vi "CRYO_MASTER_FULL_RUN3.vi"() -> ()   [LabVIEW 2017] (continued)
  T14 = enum16{"N.C.", "T3He1-1", "T3He1-2", "T3He1-3", "T3He1-4", "T3He2-1", "T3He2-2", "T3He3", "T3He4", "T3He5", "T3He6-1", "T3He6-2", "T3He7-1", "T3He7-2", "T3He8", "T3He9", "T3He10", "T4He1", "T4He2-1", "T4He2-2", "T4He3-1", "T4He3-2", "T4He3-3", "T4He3-4", "T4He4", "T4He5", "T4He6", "T4He7", "T4He8", "T4He9", "T4He10", "T1K1", "T1K2", "T1K3-1", "T1K3-2", "T1K4", "T1K5", "T1K6", "TIP1", "TIP2", "TIP3", "TIP4", "TIP5", "TIP6", "TIP7", "TTH1", "TTH2", "TTH3", "TTH4"}
  T15 = cluster{"Source":enum16{"USB6210", "USB6218AI", "USB6218AO", "LSI218", "LSI336", "DMMs"}, "SourceLabel":string}
  T16 = cluster{"Source":enum16{"USB6210", "USB6218AI", "USB6218AO", "LSI218", "LSI336", "DMMs"}, "SourceLabel":string, "FileFormat":string}[]
  T17 = cluster{"LSIName":string, "Active?":bool, "LastData":dbl[], "Labels":string[]}[]
  T18 = enum16{"N.C.", "T3He1-1", "T3He1-2", "T3He1-3", "T3He1-4", "T3He2-1", "T3He2-2", "T3He3", "T3He4", "T3He5", "T3He6-1", "T3He6-2", "T3He7-1", "T3He7-2", "T3He8", "T3He9", "T3He10", "T4He1", "T4He2-1", "T4He2-2", "T4He3-1", "T4He3-2", "T4He3-3", "T4He3-4", "T4He4", "T4He5", "T4He6", "T4He7", "T4He8", "T4He9", "T4He10", "T1K1", "T1K2", "T1K3-1", "T1K3-2", "T1K4", "T1K5", "T1K6", "TIP1", "TIP2", "TIP3", "TIP4", "TIP5", "TIP6", "TIP7", "TTH1", "TTH2", "TTH3", "TTH4"}[]
  T19 = cluster{"TimeArray (USB6218)":timestamp[], "DataArrayConv (USB6218)":dbl[]}
  T20 = cluster{"appended array":timestamp[], "ActualCurrentArray":dbl[]}
  T21 = cluster{"appended array":timestamp[], "SetCurrentArray":dbl[]}
  T22 = cluster{"appended array":timestamp[], "SetCurrentArray":dbl[]}[]
  T23 = typedef "imagedata.ctl" = cluster{"image type":i32, "image depth":i32, "image":u8[], "mask":u8[], "colors":u32[], "Rectangle":cluster{"left":i16, "top":i16, "right":i16, "bottom":i16}}
  T24 = enum16{"open", "replace", "create", "open or create", "replace or create", "replace or create with confirmation"}
  T25 = cluster{"TimeArray":timestamp[], "DataArrayConv":dbl[]}[]
  T26 = cluster{"IndexArray":i64[], "TimeArray":timestamp[], "DataArrayRaw":dbl[][], "DataArrayConv":dbl[][], "LDArray":dbl[]}
  T27 = cluster{"InstName":string, "Active?":bool, "Status":enum16{"Intialized", "Ready", "Measuring", "Terminated"}, "Labels":string[], "LabelLD":string, "FileFormat":string[], "FileFormatLD":string, "ReadLeakDet?":bool}
  T28 = cluster{"AOUT Labels[0]":string, "AOUT Labels[1]":string, "AOUT Labels[2]":string, "AOUT Labels[3]":string, "AOUT Labels[4]":string, "AOUT Labels[5]":string, "AOUT Labels[6]":string, "AOUT Labels[7]":string, "AOUT Labels[8]":string}
  T29 = cluster{"LastTimeArray":timestamp[], "LastDataArray":dbl[]}
  T30 = cluster{"LastTimeArray":timestamp[], "LastDataArray":dbl[]}[]
  T31 = cluster{"TimeArray":timestamp[], "DataArrayConv":dbl[]}
  T32 = cluster{"TimeArray":timestamp[], "DataArrayConv (USB6218)":dbl[]}
  T33 = cluster{"TimeArray":timestamp[], "M.A. Array":dbl[]}
  T34 = cluster{"TimeArray":timestamp[], "M.A. Array":dbl[]}[]
  T35 = cluster{"TimeArray":timestamp[], "DataArray":dbl[]}
  T36 = enum16{"USB6210", "USB6218AI", "USB6218AO", "LSI218", "LSI336", "DMMs"}
diagram:
  w17 = TRUE ("create if not found? (T)")
  w21 = errorcluster {"status"=FALSE, "code"=0, "source"=""} ("error in (no error)")
  w6 = errorcluster {"status"=FALSE, "code"=0, "source"=""} ("error in (no error)")
  n1 = while {
    shift-right: [w44] -> _
    shift-left: dbl[] [] -> [w50]
    shift-right: [w47] -> _
    shift-left: timestamp[] [] -> [w49]
    i -> [w48]
    stop <- w51 stop-if-true
    n2 = Wait (ms)(milliseconds to wait=u32 225) -> ()  [unwired: 1 out]
    n3 = event shown="[6] \"OUTPUT (PWR)\", \"OUTPUT (PMC)\": Value Change" {
      selector: _ -> [_ _ _ _ _ _ _]
      dyn-events: _ -> [_ _ _ _ _ _ _]
      timeout: _ -> [_ _ _ _ _ _ _]
      tunnel: [_ TRUE _ _ _ _ _] -> w51
      tunnel: w48 -> [_ _ _ _ w132 _ _]
      tunnel: [_ _ _ _ w131 w215 _] -> w44
      tunnel: w50 -> [_ _ _ _ w128 w215 _]
      tunnel: [w53 w63 _ _ w130 w214 w218] -> w47
      tunnel: w49 -> [w53 w63 _ _ w129 w214 w218]
      tunnel: w48 -> [_ _ w69 w93 _ _ w219]
      tunnel: [_ _ _ _ w119 _ _] -> w43
      event Timeout {
        n4 = event-data() -> ()  [unwired: 1 in, 3 out]
      }
      event "Stop Button": Value Change {
        w54 = FALSE
        n5 = event-data() -> ()  [unwired: 1 in, 3 out]
        n6 = local read "error out (USB6210/6218 DOUT)"() -> (w62:errorcluster)
        n7 = local read "error out (USB6210/6218 AOUT)"() -> (w59:errorcluster)
        n8 = local read "DOUT task out"() -> (w58:refnum<k21>)
        n9 = local read "AO task out"() -> (w65:refnum<k21>)
        n10 = property on="OUTPUT\n(PWR)" class="Bool (strict)"("Value"=w54) -> ()  [unwired: 2 in, 2 out]
        n11 = property on="V2 (N.C.)" class="Bool (strict)"("Val(Sgnl)"=w54) -> ()  [unwired: 2 in, 2 out]
        n12 = property on="OUTPUT\n(PMC)" class="Bool (strict)"("Value"=w54) -> ()  [unwired: 2 in, 2 out]
        n13 = Build Array(w54, w54, w54, w54) -> (w61:bool[])
        n14 = Not(x=w54) -> (.not. x?=w55:bool)
        n15 = call <vilib>:"DAQmx Clear Task.vi"("task in"=w65, "error in"=w59) -> ("error out"=w64:errorcluster)  [unwired: 13 in]
        n16 = property on="V1 (N.O.)" class="Bool (strict)"("Val(Sgnl)"=w55) -> ()  [unwired: 2 in, 2 out]
        n17 = call <vilib>:"DAQmx Write (Digital 1D Bool NChan 1Samp 1Line).vi"("task/channels in"=w58, "data"=w61, "timeout"=10.0, "error in"=w62) -> ("task out"=w57:refnum<k21>, "error out"=w56:errorcluster)  [unwired: 9 in, 1 out]
        n18 = call <vilib>:"DAQmx Clear Task.vi"("task in"=w57, "error in"=w56) -> ("error out"=w66:errorcluster)  [unwired: 13 in]
        n19 = local write "error out (USB6210/6218 AOUT)"(w64) -> ()
        n20 = local write "error out (USB6210/6218 DOUT)"(w66) -> ()
      }
      event "V1 (N.O.)": Value Change {
        n21 = event-data() -> ()  [unwired: 1 in, 3 out]
        n22 = local read "Cycle #"() -> (w72:u32)
        n23 = Greater?(x=w72, y=u32 0) -> (0:w70:bool)
        n24 = case shown="True" w70 {
          tunnel: "V1 (N.O.)" -> [_ w86]
          tunnel: w69 -> [_ w81]
          frame False {
          }
          frame True {
            n25 = Not(x=w86) -> (.not. x?=w88:bool)
            n26 = property on="OUTPUT\n(PMC)" class="Bool (strict)"() -> ("Value"=w73:bool)  [unwired: 2 in, 2 out]
            n27 = local read "error out (USB6210/6218 DOUT)"() -> (w87:errorcluster)
            n28 = property on="OUTPUT\n(PWR)" class="Bool (strict)"() -> ("Value"=w84:bool)  [unwired: 2 in, 2 out]
            n29 = property on="V2 (N.C.)" class="Bool (strict)"() -> ("Value"=w85:bool)  [unwired: 2 in, 2 out]
            n30 = local read "DOUT task out"() -> (w91:refnum<k21>)
            n31 = Build Array(w88, w85, w84, w73) -> (w77:bool[])
            n32 = local read "File Refn USB DO"() -> (w82:refnum<file>)
            n33 = Boolean To (0,1)(Boolean=w77) -> (0, 1=w76:i16[])
            n34 = Initialize Array("%d" ("element"), 3 ("dimension size")) -> (w80:string[])
            n35 = call <vilib>:"DAQmx Write (Digital 1D Bool NChan 1Samp 1Line).vi"("task/channels in"=w91, "data"=w77, "timeout"=10.0, "error in"=w87) -> ("task out"=w89:refnum<k21>, "error out"=w75:errorcluster)  [unwired: 9 in, 1 out]
            n36 = local write "DOUT task out"(w89) -> ()
            n37 = Get Date/Time In Seconds() -> (seconds since 1Jan1904=w83:timestamp)
            n38 = call "FileWrite.vi"("DataArray"=w76, "Time Stamp"=w83, "Error In"=w75, "FileFormat"=w80, "Index"=w81, "refnum in"=w82) -> ("Error Out"=w74:errorcluster)  [unwired: 4 in, 1 out]
            n39 = local write "error out (USB6210/6218 DOUT)"(w74) -> ()
          }
        }
        "V1" <- "V1 (N.O.)"
      }
      event "V2 (N.C.)": Value Change {
        n40 = event-data() -> ()  [unwired: 1 in, 3 out]
        n41 = local read "Cycle #"() -> (w96:u32)
        n42 = Greater?(x=w96, y=u32 0) -> (0:w94:bool)
        n43 = case shown="True" w94 {
          tunnel: "V2 (N.C.)" -> [_ w111]
          tunnel: w93 -> [_ w103]
          frame False {
          }
          frame True {
            n44 = property on="OUTPUT\n(PMC)" class="Bool (strict)"() -> ("Value"=w97:bool)  [unwired: 2 in, 2 out]
            n45 = property on="V1 (N.O.)" class="Bool (strict)"() -> ("Value"=w110:bool)  [unwired: 2 in, 2 out]
            n46 = Not(x=w110) -> (.not. x?=w109:bool)
            n47 = local read "error out (USB6210/6218 DOUT)"() -> (w114:errorcluster)
            n48 = property on="OUTPUT\n(PWR)" class="Bool (strict)"() -> ("Value"=w108:bool)  [unwired: 2 in, 2 out]
            n49 = local read "DOUT task out"() -> (w115:refnum<k21>)
            n50 = Build Array(w109, w111, w108, w97) -> (w106:bool[])
            n51 = local read "File Refn USB DO"() -> (w107:refnum<file>)
            n52 = Boolean To (0,1)(Boolean=w106) -> (0, 1=w105:i16[])
            n53 = Initialize Array("%d" ("element"), 3 ("dimension size")) -> (w100:string[])
            n54 = call <vilib>:"DAQmx Write (Digital 1D Bool NChan 1Samp 1Line).vi"("task/channels in"=w115, "data"=w106, "timeout"=10.0, "error in"=w114) -> ("task out"=w112:refnum<k21>, "error out"=w99:errorcluster)  [unwired: 9 in, 1 out]
            n55 = local write "DOUT task out"(w112) -> ()
            n56 = Get Date/Time In Seconds() -> (seconds since 1Jan1904=w104:timestamp)
            n57 = call "FileWrite.vi"("DataArray"=w105, "Time Stamp"=w104, "Error In"=w99, "FileFormat"=w100, "Index"=w103, "refnum in"=w107) -> ("Error Out"=w98:errorcluster)  [unwired: 4 in, 1 out]
            n58 = local write "error out (USB6210/6218 DOUT)"(w98) -> ()
          }
        }
        "V2" <- "V2 (N.C.)"
      }
      event "Set Current (mA)\n (PMC)", "Set Current (mA)\n (PWR)", "update current": Value Change {
        n59 = event-data() -> ()  [unwired: 1 in, 3 out]
        n60 = case shown="True" "CONTROL KIKUSUI?" {
          tunnel: w132 -> [_ w183]
          tunnel: [w142 w176] -> w131
          tunnel: [w145 w175] -> w130
          tunnel: w129 -> [w147 w178]
          tunnel: w128 -> [w143 w177]
          tunnel: "Set Current (mA)\n (PWR)" -> [_ w155]
          tunnel: "Set Current (mA)\n (PMC)" -> [_ w159]
          frame False {
            w144 = 0.0 ("element")
            n61 = Get Date/Time In Seconds() -> (seconds since 1Jan1904=w146:timestamp)
            n62 = local read "AO task out"() -> (w152:refnum<k21>)
            n63 = Build Array (concatenate)(w147, w146) -> (w145:timestamp[])
            n64 = Build Array (concatenate)(w143, w144) -> (w142:dbl[])
            n65 = Build Array(w144, w144) -> (w150:dbl[])
            n66 = call <vilib>:"DAQmx Write (Analog 1D DBL NChan 1Samp).vi"("task/channels in"=w152, "data"=w150, "timeout"=100.0, "error in"=errorcluster {"status"=FALSE, "code"=0, "source"=""}) -> ("task out"=w153:refnum<k21>, "error out"=w148:errorcluster)  [unwired: 9 in, 1 out]
            n67 = local write "AO task out"(w153) -> ()
            n68 = local write "error out (KIKUSI CTRL)"(w148) -> ()
          }
          frame True {
            w170 = 2 ("index")
            n69 = xnode "Formula"("X1"=w155) -> ("Result"=w172:dbl)  [unwired: 1 in, 1 out]
            n70 = xnode "Formula"("X1"=w159) -> ("Result"=w166:dbl)  [unwired: 1 in, 1 out]
            n71 = Build Array (concatenate)(w177, w155) -> (w176:dbl[])
            n72 = In Range and Coerce(upper limit=10.0, x=w172, lower limit=0.0 ("y")) -> (coerced(x)=w164:dbl, In Range?=w165:bool)
            n73 = In Range and Coerce(upper limit=10.0, x=w166, lower limit=0.0 ("y")) -> (coerced(x)=w161:dbl, In Range?=w162:bool)
            n74 = case shown="False" w165 {
              tunnel: w164 -> [_ w195]
              tunnel: [0.0 ("upper limit") w195] -> w163
              frame False {
              }
              frame True {
              }
            }
            n75 = case shown="True" w162 {
              tunnel: w161 -> [_ w193]
              tunnel: [0.0 ("upper limit") w193] -> w160
              frame False {
              }
              frame True {
              }
            }
            n76 = Multiply(x=w155, y=0.001) -> (x*y=w154:dbl)
            n77 = Multiply(x=w159, y=0.001) -> (x*y=w158:dbl)
            n78 = local read "File Refn USB AO"() -> (w184:refnum<file>)
            n79 = Build Array(w154, w158, w163, w160) -> (w171:dbl[])
            "USB 6218 AOUT" <- w171
            n80 = Initialize Array("%.3f", 4 ("dimension size")) -> (w185:string[])
            n81 = Get Date/Time In Seconds() -> (seconds since 1Jan1904=w179:timestamp)
            n82 = local read "AO task out"() -> (w189:refnum<k21>)
            n83 = call "FileWrite.vi"("DataArray"=w171, "Time Stamp"=w179, "Error In"=errorcluster {"status"=FALSE, "code"=0, "source"=""} ("error in"), "FileFormat"=w185, "Index"=w183, "refnum in"=w184) -> ("Error Out"=w181:errorcluster, "Byte Stream File Refnum"=w180:refnum<file>)  [unwired: 4 in]
            n84 = Build Array (concatenate)(w178, w179) -> (w175:timestamp[])
            n85 = Array Subset(array=w171, index=w170, length=w170) -> (w169:dbl[])
            n86 = local write "File Refn USB AO"(w180) -> ()
            n87 = call <vilib>:"DAQmx Write (Analog 1D DBL NChan 1Samp).vi"("task/channels in"=w189, "data"=w169, "timeout"=100.0, "error in"=w181) -> ("task out"=w190:refnum<k21>, "error out"=→"error out (KIKUSI CTRL)":errorcluster)  [unwired: 9 in, 1 out]
            n88 = local write "AO task out"(w190) -> ()
          }
        }
        n89 = local read "All Labels (USB6218)"() -> (w125:string[])
        n90 = local read "DataArrayConv (USB6218)"() -> (w124:dbl[][])
        n91 = local read "Last Data \n(USB6218)"() -> (w121:dbl[])
        n92 = local read "TimeArray (USB6218)"() -> (w122:timestamp[])
        n93 = Search 1D Array(1D array=w125, element="I_CV") -> (index of element=w126:i32)  [unwired: 1 in]
        n94 = Index Array(array=w124, index (row)=w126) -> (element=w123:dbl[])  [unwired: 1 in]
        n95 = Index Array(array=w121, index=w126) -> (element=w118:dbl)
        n96 = Bundle("TimeArray (USB6218)"=w122, "DataArrayConv (USB6218)"=w123) -> (w119:T19)  [unwired: 1 in]
        n97 = xnode "Formula"("X1"=w118) -> ("Result"=→"Monitor Current (mA)":dbl)  [unwired: 1 in, 1 out]
      }
      event "upper limit (mA)\n (PWR)", "lower limit (mA) \n(PWR)": Value Change {
        n98 = event-data() -> ()  [unwired: 1 in, 6 out]
        n99 = property on="Set Current (mA)\n (PWR)" class="DigNum (strict)"("Maximum"="upper limit (mA)\n (PWR)", "Minimum"="lower limit (mA) \n(PWR)") -> ()  [unwired: 2 in, 2 out]
        n100 = property on="Set Current (mA)\n (PMC)" class="DigNum (strict)"("Maximum"="upper limit (mA)\n (PMC)", "Minimum"="lower limit (mA) \n(PMC)") -> ()  [unwired: 2 in, 2 out]
      }
      event "OUTPUT\n(PWR)", "OUTPUT\n(PMC)": Value Change {
        n101 = event-data() -> ()  [unwired: 1 in, 6 out]
        n102 = local read "Cycle #"() -> (w222:u32)
        n103 = Greater?(x=w222, y=u32 0) -> (0:w220:bool)
        n104 = case shown="True" w220 {
          tunnel: w219 -> [_ w227]
          frame False {
          }
          frame True {
            n105 = property on="V1 (N.O.)" class="Bool (strict)"() -> ("Value"=w238:bool)  [unwired: 2 in, 2 out]
            n106 = Not(x=w238) -> (.not. x?=w237:bool)
            n107 = local read "error out (USB6210/6218 DOUT)"() -> (w241:errorcluster)
            n108 = property on="V2 (N.C.)" class="Bool (strict)"() -> ("Value"=w236:bool)  [unwired: 2 in, 2 out]
            n109 = local read "DOUT task out"() -> (w242:refnum<k21>)
            n110 = Build Array(w237, w236, "OUTPUT\n(PWR)", "OUTPUT\n(PMC)") -> (w225:bool[])
            n111 = local read "File Refn USB DO"() -> (w228:refnum<file>)
            n112 = Boolean To (0,1)(Boolean=w225) -> (0, 1=w224:i16[])
            n113 = call <vilib>:"DAQmx Write (Digital 1D Bool NChan 1Samp 1Line).vi"("task/channels in"=w242, "data"=w225, "timeout"=10.0, "error in"=w241) -> ("task out"=w239:refnum<k21>, "error out"=w232:errorcluster)  [unwired: 9 in, 1 out]
            n114 = Initialize Array("%d" ("element"), 3 ("dimension size")) -> (w230:string[])
            n115 = local write "DOUT task out"(w239) -> ()
            n116 = Get Date/Time In Seconds() -> (seconds since 1Jan1904=w229:timestamp)
            n117 = call "FileWrite.vi"("DataArray"=w224, "Time Stamp"=w229, "Error In"=w232, "FileFormat"=w230, "Index"=w227, "refnum in"=w228) -> ("Error Out"=w231:errorcluster, "Byte Stream File Refnum"=w226:refnum<file>)  [unwired: 4 in]
            n118 = local write "File Refn USB DO"(w226) -> ()
            n119 = local write "error out (USB6210/6218 DOUT)"(w231) -> ()
          }
        }
      }
    }
    n120 = Bundle(w47, w44) -> (w46:cluster{timestamp[], dbl[]})  [unwired: 1 in]
    n121 = Build Array(w46, w43) -> (→"Graph 7":T10)
  }
  n122 = while {
    shift-right: [w251] -> _
    shift-left: refnum<class "6240AData.lvclass"> refnum ("6240AData.lvclass") -> [w249]
    shift-right: [w247] -> _
    shift-left: errorcluster {"status"=FALSE, "code"=0, "source"=""} ("error in (no error)") -> [w248]
    i -> [w243]
    stop <- w250 stop-if-true
    n123 = Wait (ms)(milliseconds to wait=u32 231) -> ()  [unwired: 1 out]
    n124 = Equal?(x=w243, y=0) -> (x = y?=w245:bool)
    n125 = case shown="True" w245 {
      frame False {
      }
      frame True {
        n126 = property on="Initialized?" class="Bool (strict)"("Val(Sgnl)"=FALSE ("Value (Signaling)")) -> ()  [unwired: 2 in, 2 out]
      }
    }
    n127 = event shown="[2] \"upper limit (mA)\", \"lower limit (mA)\": Value Change" {
      selector: _ -> [_ _ _ _ _]
      dyn-events: _ -> [_ _ _ _ _]
      timeout: _ -> [_ _ _ _ _]
      tunnel: [w254 w269 _ w318 w339] -> w251
      tunnel: [_ _ _ _ TRUE ("Value (Signaling)")] -> w250
      tunnel: w249 -> [w254 w268 _ w302 w337]
      tunnel: w248 -> [w253 w267 _ w301 w335]
      tunnel: [w253 w266 _ w316 w338] -> w247
      tunnel: w243 -> [_ w265 _ _ _]
      tunnel: w243 -> [_ _ _ w310 _]
      event Timeout {
        n128 = event-data() -> ()  [unwired: 1 in, 3 out]
      }
      event "update values", "SetCurrent 1 (mA)", "SetCurrent 2 (mA)": Value Change {
        w258 = 1000.0 ("y")
        n129 = event-data() -> ()  [unwired: 1 in, 6 out]
        n130 = local read "Initialized?"() -> (w264:bool)
        n131 = Divide(x="SetCurrent 1 (mA)", y=w258) -> (x/y=w259:dbl)
        n132 = Divide(x="SetCurrent 2 (mA)", y=w258) -> (x/y=w260:dbl)
        n133 = Build Array(w259, w260) -> (w257:dbl[])
        n134 = Not Equal?(x=w264, y=FALSE) -> (x != y?=w262:bool)
        n135 = case shown="True" w262 {
          tunnel: [w271 w295] -> w269
          tunnel: "Output\n (ADCMT)" -> [_ w294]
          tunnel: w268 -> [w271 w293]
          tunnel: w267 -> [w270 w292]
          tunnel: [w270 w291] -> w266
          tunnel: w265 -> [_ w287]
          tunnel: w257 -> [_ w273]
          frame False {
          }
          frame True {
            w280 = 1 ("index (col)")
            w281 = 0 ("disabled index (col)")
            n136 = call-dynamic "6240AData_execute.vi"("6240AData in"=w293, "SetCurrent (A)"=w273, "FileFormat"="%3.5f", "Output status"=w294, "ExecutionIndex"=w287, "error in (no error)"=w292) -> ("ActualVoltage (V)"=w272:dbl[], "ActualCurrent (A)"=w286:dbl[], "6240AData out"=w295:refnum<class "6240AData.lvclass">, "appended array"=w276:timestamp[], "SetCurrentArray"=w282:dbl[][], "ActualCurrentArray"=w289:dbl[][], "error out"=w291:errorcluster)  [unwired: 3 in]
            n137 = property on="ActualVoltage (V)" class="Arr (strict)"("Val(Sgnl)"=w272) -> ()  [unwired: 2 in, 2 out]
            n138 = property on="ActualCurrent (A)" class="Arr (strict)"("Val(Sgnl)"=w286) -> ()  [unwired: 2 in, 2 out]
            n139 = Index Array(array=w289, index (col) #1=w281, index (col) #2=w280) -> (element #1=w290:dbl[], element #2=w284:dbl[])  [unwired: 2 in]
            n140 = Index Array(array=w282, index (col) #1=w281, index (col) #2=w280) -> (element #1=w278:dbl[], element #2=w275:dbl[])  [unwired: 2 in]
            n141 = Bundle("appended array"=w276, "ActualCurrentArray"=w290) -> (w285:T20)  [unwired: 1 in]
            n142 = Bundle("appended array"=w276, "ActualCurrentArray"=w284) -> (w279:T20)  [unwired: 1 in]
            n143 = Bundle("appended array"=w276, "SetCurrentArray"=w278) -> (w277:T21)  [unwired: 1 in]
            n144 = Bundle("appended array"=w276, "SetCurrentArray"=w275) -> (w274:T21)  [unwired: 1 in]
            n145 = Build Array(w285, w279, w277, w274) -> (→"Graph 6":T22)
          }
        }
      }
      event "upper limit (mA)", "lower limit (mA)": Value Change {
        n146 = event-data() -> ()  [unwired: 1 in, 6 out]
        n147 = property on="SetCurrent 1 (mA)" class="DigNum (strict)"("Maximum"="upper limit (mA)", "Minimum"="lower limit (mA)") -> ()  [unwired: 2 in, 2 out]
        n148 = property on="SetCurrent 2 (mA)" class="DigNum (strict)"("Maximum"="upper limit (mA)", "Minimum"="lower limit (mA)") -> ()  [unwired: 2 in, 2 out]
      }
      event "Initialize": Value Change {
        w312 = FALSE
        n149 = event-data() -> ()  [unwired: 1 in, 6 out]
        n150 = local read "Initialized?"() -> (w300:bool)
        n151 = case shown="True" w300 {
          tunnel: w302 -> [w328 w332]
          tunnel: w301 -> [w327 w331]
          tunnel: [w328 w330] -> w299
          tunnel: [w327 w329] -> w298
          frame False {
          }
          frame True {
            n152 = call-dynamic "6240AData_terrminate.vi"("error in (no error)"=w331, "6240AData in"=w332) -> ("error out"=w329:errorcluster, "6240AData out"=w330:refnum<class "6240AData.lvclass">)  [unwired: 8 in]
          }
        }
        n153 = property on="Initialized?" class="Bool (strict)"("Val(Sgnl)"=TRUE ("Value (Signaling)")) -> ()  [unwired: 2 in, 2 out]
        n154 = local read "SetCurrent 2 (mA)"() -> (w305:dbl)
        n155 = local read "SetCurrent 1 (mA)"() -> (w308:dbl)
        n156 = local read "RUN Identifier"() -> (w320:string)
        n157 = local read "Base Path"() -> (w321:path)
        n158 = Divide(x=w308, y=1000.0) -> (x/y=w307:dbl)
        n159 = Divide(x=w305, y=1000.0) -> (x/y=w304:dbl)
        n160 = Get Date/Time In Seconds() -> ()  [unwired: 1 out]
        n161 = call-dynamic "6240AData_initialize.vi"("6240AData in"=w299, "RunIdentifier"=w320, "InstName"="InstName", "base path"=w321, "VISA"="VISA", "error in (no error)"=w298, "CtrlLabels"="CtrlLabels", "Voltage limits (V)"="Voltage limits (V)") -> ("6240AData out"=w319:refnum<class "6240AData.lvclass">, "error out"=w317:errorcluster)  [unwired: 6 in]
        n162 = Build Array(w307, w304) -> (w303:dbl[])
        n163 = Build Array(w312, w312) -> (w311:bool[])
        n164 = call-dynamic "6240AData_execute.vi"("6240AData in"=w319, "SetCurrent (A)"=w303, "FileFormat"="%3.5f", "Output status"=w311, "ExecutionIndex"=w310, "error in (no error)"=w317) -> ("ActualVoltage (V)"=w314:dbl[], "ActualCurrent (A)"=w313:dbl[], "6240AData out"=w318:refnum<class "6240AData.lvclass">, "error out"=w316:errorcluster)  [unwired: 3 in, 3 out]
        n165 = property on="ActualVoltage (V)" class="Arr (strict)"("Val(Sgnl)"=w314) -> ()  [unwired: 2 in, 2 out]
        n166 = property on="ActualCurrent (A)" class="Arr (strict)"("Val(Sgnl)"=w313) -> ()  [unwired: 2 in, 2 out]
      }
      event "Stop Button": Value Change {
        n167 = event-data() -> ()  [unwired: 1 in, 6 out]
        n168 = local read "Initialized?"() -> (w333:bool)
        n169 = case shown="False" w333 {
          tunnel: w337 -> [w342 w354]
          tunnel: [w342 w353] -> w336
          tunnel: w335 -> [w341 w352]
          tunnel: [w341 w351] -> w334
          frame False {
          }
          frame True {
            w358 = FALSE
            n170 = local read "SetCurrent 2 (mA)"() -> (w344:dbl)
            n171 = local read "SetCurrent 1 (mA)"() -> (w348:dbl)
            n172 = Divide(x=w348, y=1000.0) -> (x/y=w346:dbl)
            n173 = Divide(x=w344, y=1000.0) -> (x/y=w343:dbl)
            n174 = Build Array(w346, w343) -> (w350:dbl[])
            n175 = Build Array(w358, w358) -> (w349:bool[])
            n176 = property on="Output\n (ADCMT)" class="Arr (strict)"("Val(Sgnl)"=w349) -> ()  [unwired: 2 in, 2 out]
            n177 = call-dynamic "6240AData_execute.vi"("6240AData in"=w354, "SetCurrent (A)"=w350, "FileFormat"="%3.5f", "Output status"=w349, "error in (no error)"=w352) -> ("ActualVoltage (V)"=w355:dbl[], "ActualCurrent (A)"=w356:dbl[], "6240AData out"=w353:refnum<class "6240AData.lvclass">, "error out"=w351:errorcluster)  [unwired: 4 in, 3 out]
            n178 = property on="ActualVoltage (V)" class="Arr (strict)"("Val(Sgnl)"=w355) -> ()  [unwired: 2 in, 2 out]
            n179 = property on="ActualCurrent (A)" class="Arr (strict)"("Val(Sgnl)"=w356) -> ()  [unwired: 2 in, 2 out]
          }
        }
        n180 = call-dynamic "6240AData_terrminate.vi"("error in (no error)"=w334, "6240AData in"=w336) -> ("error out"=w338:errorcluster, "6240AData out"=w339:refnum<class "6240AData.lvclass">)  [unwired: 8 in]
      }
    }
    "error out (ADCMT6420A)" <- w247
  }
  n181 = while {
    stop <- w367 stop-if-true
    n182 = Get Date/Time In Seconds() -> (seconds since 1Jan1904=w366:timestamp)
    n183 = Format Date/Time String(time format string (%c)="%Y%m", seconds (now)=w366) -> (date/time string=w363:string)  [unwired: 1 in]
    n184 = Build Path(base path="Base Path (screenshots)", name or relative path=w363) -> (appended path=w362:path)
    n185 = Create Folder(path (use dialog)=w362, error in=errorcluster {"status"=FALSE, "code"=0, "source"=""}) -> (created path=w359:path, error out=→"error out (monthly folder creation)":errorcluster)  [unwired: 1 in, 1 out]
    n186 = event shown="[1] \"Frontpanel screenshots\": Value Change" {
      selector: _ -> [_ _ _]
      dyn-events: _ -> [_ _ _]
      timeout: _ -> [_ _ _]
      tunnel: [FALSE _ TRUE] -> w367
      tunnel: w359 -> [_ w375 _]
      tunnel: w366 -> [_ w374 _]
      event Timeout {
        n187 = event-data() -> ()  [unwired: 1 in, 3 out]
      }
      event "Frontpanel screenshots": Value Change {
        n188 = event-data() -> ()  [unwired: 1 in, 3 out]
        n189 = property class="TabCtl (strict)"() -> ("Value"=w372:T1)  [unwired: 2 in, 2 out]
        n190 = stacked-sequence {
          tunnel: w375 -> [w381 w403 w425 w447 w469 w491 w513 w535 w557 _]
          tunnel: w374 -> [w380 w402 w424 w446 w468 w490 w512 w534 w556 _]
          tunnel: [w378 _ _ _ _ _ _ _ _ _] -> w373
          tunnel: w372 -> [w377 _ _ _ _ _ _ _ _ _]
          tunnel: [w377 _ _ _ _ _ _ _ _ _] -> w371
          tunnel: "cryostatus_" ("string") -> [w376 w399 w421 w443 w465 w487 w509 w531 w553 _]
          frame #0 {
            n191 = flat-sequence {
              tunnel: w380 -> [w383]
              tunnel: [w383] -> w379
              tunnel: w381 -> [w398]
              tunnel: w379 -> [w386]
              tunnel: [w385] -> w378
              tunnel: w376 -> [w384]
              frame #0 {
                n192 = property class="TabCtl (strict)"("Val(Sgnl)"=T1."NI USB CONFIG" ("Value (Signaling)")) -> ()  [unwired: 2 in, 2 out]
              }
              frame #1 {
                w396 = "_" ("string")
                n193 = local read "Cycle #"() -> (w394:u32)
                n194 = call "LV_UNIXTIME.vi"("current time"=w386) -> ("date/time string"=w397:string)  [unwired: 9 in, 1 out]
                n195 = Format Value(format string="%06d", value (0)=w394) -> (output string=w393:string)  [unwired: 1 in]
                n196 = Concatenate Strings(w384, w397, w396, w393, w396, "page1.png" ("string")) -> (w391:string)
                n197 = invoke class="TabCtl (strict)" method="Get Image"(error in=errorcluster {"status"=FALSE, "code"=0, "source"=""} ("error in (no error)")) -> (error out=w387:errorcluster, "image data"=w389:T23)  [unwired: 5 in, 4 out]
                n198 = Build Path(base path=w398, name or relative path=w391) -> (appended path=w390:path)
                n199 = call <vilib>:"Write PNG File.vi"("error in (no error)"=w387, "image data"=w389, "path to PNG file"=w390) -> ("error out"=w385:errorcluster)  [unwired: 7 in, 1 out]
              }
            }
          }
          frame #1 {
            n200 = flat-sequence {
              tunnel: w402 -> [w405]
              tunnel: [w405] -> w401
              tunnel: w403 -> [w420]
              tunnel: w401 -> [w408]
              tunnel: [w407] -> w400
              tunnel: w399 -> [w406]
              frame #0 {
                n201 = property class="TabCtl (strict)"("Val(Sgnl)"=T1."NI USB CONFIG" ("Value (Signaling)")) -> ()  [unwired: 2 in, 2 out]
              }
              frame #1 {
                w418 = "_" ("string")
                n202 = local read "Cycle #"() -> (w416:u32)
                n203 = call "LV_UNIXTIME.vi"("current time"=w408) -> ("date/time string"=w419:string)  [unwired: 9 in, 1 out]
                n204 = Format Value(format string="%06d", value (0)=w416) -> (output string=w415:string)  [unwired: 1 in]
                n205 = Concatenate Strings(w406, w419, w418, w415, w418, "page2.png" ("string")) -> (w413:string)
                n206 = invoke class="TabCtl (strict)" method="Get Image"(error in=errorcluster {"status"=FALSE, "code"=0, "source"=""} ("error in (no error)")) -> (error out=w409:errorcluster, "image data"=w411:T23)  [unwired: 5 in, 4 out]
                n207 = Build Path(base path=w420, name or relative path=w413) -> (appended path=w412:path)
                n208 = call <vilib>:"Write PNG File.vi"("error in (no error)"=w409, "image data"=w411, "path to PNG file"=w412) -> ("error out"=w407:errorcluster)  [unwired: 7 in, 1 out]
              }
            }
            n209 = local write "error out (frontpanel screenshots)"(w400) -> ()
          }
          frame #2 {
            n210 = flat-sequence {
              tunnel: w424 -> [w427]
              tunnel: [w427] -> w423
              tunnel: w425 -> [w442]
              tunnel: w423 -> [w430]
              tunnel: [w429] -> w422
              tunnel: w421 -> [w428]
              frame #0 {
                n211 = property class="TabCtl (strict)"("Val(Sgnl)"=T1."NI USB CONFIG" ("Value (Signaling)")) -> ()  [unwired: 2 in, 2 out]
              }
              frame #1 {
                w440 = "_" ("string")
                n212 = local read "Cycle #"() -> (w438:u32)
                n213 = Format Value(format string="%06d", value (0)=w438) -> (output string=w437:string)  [unwired: 1 in]
                n214 = call "LV_UNIXTIME.vi"("current time"=w430) -> ("date/time string"=w441:string)  [unwired: 9 in, 1 out]
                n215 = Concatenate Strings(w428, w441, w440, w437, w440, "page3.png" ("string")) -> (w435:string)
                n216 = invoke class="TabCtl (strict)" method="Get Image"(error in=errorcluster {"status"=FALSE, "code"=0, "source"=""} ("error in (no error)")) -> (error out=w431:errorcluster, "image data"=w433:T23)  [unwired: 5 in, 4 out]
                n217 = Build Path(base path=w442, name or relative path=w435) -> (appended path=w434:path)
                n218 = call <vilib>:"Write PNG File.vi"("error in (no error)"=w431, "image data"=w433, "path to PNG file"=w434) -> ("error out"=w429:errorcluster)  [unwired: 7 in, 1 out]
              }
            }
            n219 = local write "error out (frontpanel screenshots)"(w422) -> ()
          }
          frame #3 {
            n220 = flat-sequence {
              tunnel: w446 -> [w449]
              tunnel: [w449] -> w445
              tunnel: w447 -> [w464]
              tunnel: w445 -> [w452]
              tunnel: [w451] -> w444
              tunnel: w443 -> [w450]
              frame #0 {
                n221 = property class="TabCtl (strict)"("Val(Sgnl)"=T1."HE AUTO FILL" ("Value (Signaling)")) -> ()  [unwired: 2 in, 2 out]
              }
              frame #1 {
                w462 = "_" ("string")
                n222 = local read "Cycle #"() -> (w460:u32)
                n223 = Format Value(format string="%06d", value (0)=w460) -> (output string=w459:string)  [unwired: 1 in]
                n224 = call "LV_UNIXTIME.vi"("current time"=w452) -> ("date/time string"=w463:string)  [unwired: 9 in, 1 out]
                n225 = Concatenate Strings(w450, w463, w462, w459, w462, "page4.png" ("string")) -> (w457:string)
                n226 = invoke class="TabCtl (strict)" method="Get Image"(error in=errorcluster {"status"=FALSE, "code"=0, "source"=""} ("error in (no error)")) -> (error out=w453:errorcluster, "image data"=w455:T23)  [unwired: 5 in, 4 out]
                n227 = Build Path(base path=w464, name or relative path=w457) -> (appended path=w456:path)
                n228 = call <vilib>:"Write PNG File.vi"("error in (no error)"=w453, "image data"=w455, "path to PNG file"=w456) -> ("error out"=w451:errorcluster)  [unwired: 7 in, 1 out]
              }
            }
            n229 = local write "error out (frontpanel screenshots)"(w444) -> ()
          }
          frame #4 {
            n230 = flat-sequence {
              tunnel: w468 -> [w471]
              tunnel: [w471] -> w467
              tunnel: w469 -> [w486]
              tunnel: w467 -> [w474]
              tunnel: [w473] -> w466
              tunnel: w465 -> [w472]
              frame #0 {
                n231 = property class="TabCtl (strict)"("Val(Sgnl)"=T1."VALVE/HEATER CTRL" ("Value (Signaling)")) -> ()  [unwired: 2 in, 2 out]